vi "NoiseTest.vi"() -> ()   [LabVIEW 2022 SP3]
panel:
  in  "Case":u16(ring) items=["Probe in Air", "Finger on Probe", "In air 2", "In air 3"]
  in  "log scale for image":bool=TRUE
  in  "Reverse Subtraction":bool
  out "Raw Data file":dbl[][](graph)
  out "Line number":dbl format="%.2f"
  out "subtraction of noise line from RF line":i16[](graph)
  out "raw RF line":i16[](graph)
  out "noise line 1":i16[](graph)
  out "noise line 2":i16[](graph)
  out "Noise Lines Subtracted":dbl[][](graph)
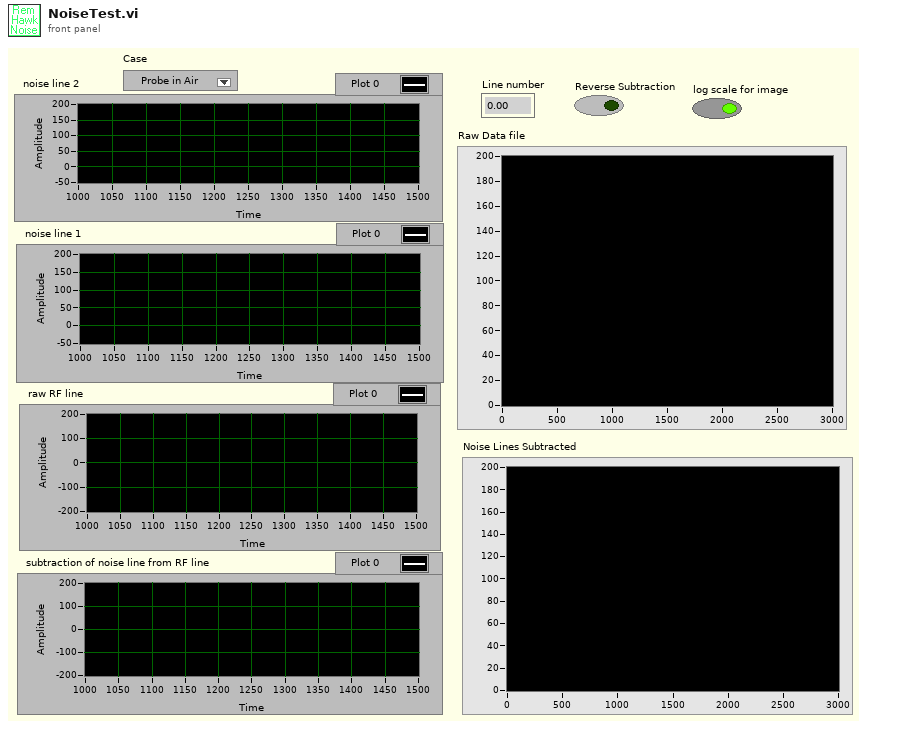
[diagram p1: front panel]
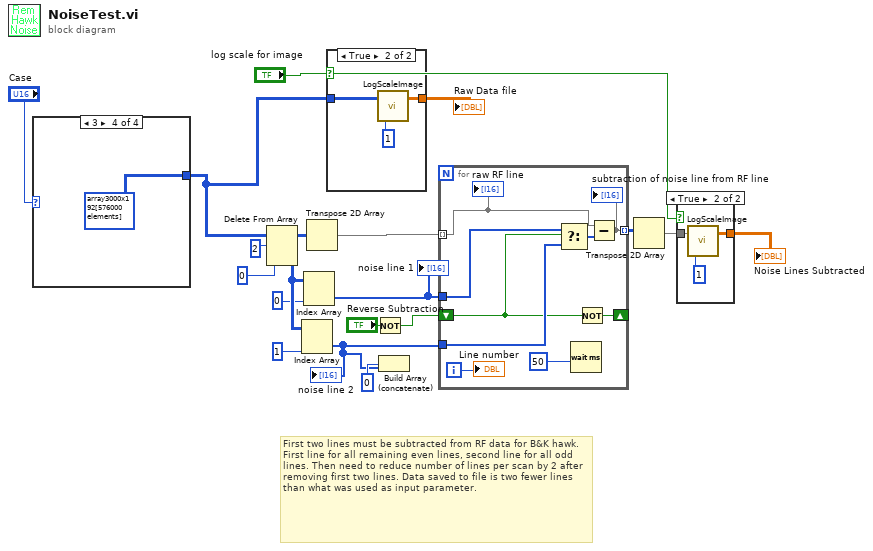
[diagram p0: block diagram]
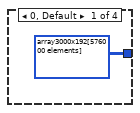
[diagram p2: hidden frame]
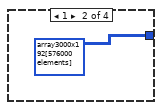
[diagram p3: hidden frame]
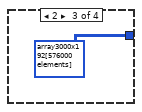
[diagram p4: hidden frame]
diagram:
  # "First two lines must be subtracted from RF data for B&K hawk. First line for all remaining even lines, second line for all odd lines. Then need to reduce number of lines per scan by 2 after removing first two lines. Data saved to file is two fewer lines than what was used as input parameter."
  n1 = case shown="3" "Case" {
    tunnel: [i16[][] array3000x192[576000 elements] ("2-D data array") i16[][] array3000x192[576000 elements] ("2-D data array") i16[][] array3000x192[576000 elements] ("2-D data array") i16[][] array3000x192[576000 elements] ("2-D data array")] -> w5
    frame 0, Default {
    }
    frame 1 {
    }
    frame 2 {
    }
    frame 3 {
    }
  }
  n2 = Delete From Array(array=w5, length=2, index (col)=0) -> (deleted portion=w15:i16[][], array with subset deleted=w18:i16[][])  [unwired: 1 in]
  n3 = Index Array(array=w15, index (col)=1) -> (element=w7:i16[])  [unwired: 1 in]
  "noise line 2" <- w7
  n4 = Index Array(array=w15, index (col)=0) -> (element=w10:i16[])  [unwired: 1 in]
  "noise line 1" <- w10
  n5 = Transpose 2D Array(2D array=w18) -> (transposed array=w16:i16[][])
  n6 = case shown="True" "log scale for image" {
    tunnel: w5 -> [w24 w26]
    tunnel: [w24 w25] -> w4
    frame False {
    }
    frame True {
      n7 = call "LogScaleImage.vi"("A/D bits"=1, "input array"=w26) -> ("log scale image"=w25:dbl[][])  [unwired: 1 out]
    }
  }
  "Raw Data file" <- w4
  n8 = Not(x="Reverse Subtraction") -> (.not. x?=w2:bool)
  n9 = Build Array (concatenate)(0, w7) -> ()  [unwired: 1 out]
  n10 = for {
    tunnel: w16 -> [w31] mode=indexing
    tunnel: w10 -> [w36]
    tunnel: w7 -> [w35]
    tunnel: [w30] -> w12 mode=indexing
    shift-right: [w32] -> _
    shift-left: w2 -> [w33]
    i -> [w28]
    n11 = Select(t=w36, s=w33, f=w35) -> (s? t:f=w34:i16[])
    n12 = Wait (ms)(milliseconds to wait=50) -> ()  [unwired: 1 out]
    n13 = Not(x=w33) -> (.not. x?=w32:bool)
    n14 = Subtract(x=w31, y=w34) -> (x-y=w30:i16[])
    "subtraction of noise line from RF line" <- w30
    "raw RF line" <- w31
    "Line number" <- w28
  }
  n15 = Transpose 2D Array(2D array=w12) -> (transposed array=w9:i16[][])
  n16 = case shown="True" "log scale for image" {
    tunnel: [w37 w40] -> w19
    tunnel: w9 -> [w37 w38]
    frame False {
    }
    frame True {
      n17 = call "LogScaleImage.vi"("A/D bits"=1, "input array"=w38) -> ("log scale image"=w40:dbl[][])  [unwired: 1 out]
    }
  }
  "Noise Lines Subtracted" <- w19
